vi "pharmaBot_v0.019.vi"() -> ()   [LabVIEW 2015] (continued)
  n42 = control-ref of="memtest 1"() -> (w236:refnum<vi>)
  n43 = control-ref of="cell stats"() -> (w235:refnum<vi>)
  n44 = control-ref of="Ra 1"() -> (w234:refnum<vi>)
  n45 = control-ref of="Ra 2"() -> (w233:refnum<vi>)
  n46 = control-ref of="Cm 1"() -> (w232:refnum<vi>)
  n47 = control-ref of="Cm 2"() -> (w231:refnum<vi>)
  n48 = control-ref of="Iholding 2"() -> (w230:refnum<vi>)
  n49 = control-ref of="P2"() -> (w229:refnum<vi>)
  n50 = control-ref of="Iholding 1"() -> (w228:refnum<vi>)
  n51 = control-ref of="P1"() -> (w227:refnum<vi>)
  n52 = control-ref of="channels to initialize"() -> (w226:refnum<vi>)
  n53 = control-ref of="Multiclamp Handle"() -> (w225:refnum<vi>)
  n54 = control-ref of="mclamp cluster"() -> (w224:refnum<vi>)
  n55 = control-ref of="manip 1 on"() -> (w223:refnum<vi>)
  n56 = control-ref of="manip 2 on"() -> (w222:refnum<vi>)
  n57 = control-ref of="daq_do 2"() -> (w244:refnum<vi>)
  n58 = control-ref of="daq_do 1"() -> (w243:refnum<vi>)
  n59 = control-ref of="NH method"() -> (w179:refnum<vi>)
  n60 = control-ref of="depth"() -> (w178:refnum<vi>)
  n61 = control-ref of="NH R"() -> (w177:refnum<vi>)
  n62 = control-ref of="start GS time 1"() -> (w176:refnum<vi>)
  n63 = control-ref of="max steps to take"() -> (w175:refnum<vi>)
  n64 = control-ref of="Pipette broken threshold (MOhms)"() -> (w173:refnum<vi>)
  n65 = control-ref of="Extra threshold (MOhms)"() -> (w172:refnum<vi>)
  n66 = control-ref of="max hunt distance (um)"() -> (w171:refnum<vi>)
  n67 = control-ref of="Neuron Detection Threshold (MOhms)"() -> (w170:refnum<vi>)
  n68 = control-ref of="hunt pressure (mBar)"() -> (w169:refnum<vi>)
  n69 = control-ref of="NH step size (steps)"() -> (w168:refnum<vi>)
  n70 = control-ref of="current cell 2"() -> (w167:refnum<vi>)
  n71 = control-ref of="cells (image px)"() -> (w166:refnum<vi>)
  n72 = control-ref of="current stage pos (steps)"() -> (w165:refnum<vi>)
  n73 = control-ref of="previous time in"() -> (w164:refnum<vi>)
  n74 = control-ref of="current cell 1"() -> (w162:refnum<vi>)
  n75 = control-ref of="breakin counter 1"() -> (w161:refnum<vi>)
  n76 = control-ref of="MAX Break In Pressure (mbar)"() -> (w160:refnum<vi>)
  n77 = control-ref of="vhold applied?"() -> (w159:refnum<vi>)
  n78 = control-ref of="time"() -> (w158:refnum<vi>)
  n79 = control-ref of="GS R"() -> (w157:refnum<vi>)
  n80 = control-ref of="Vholding (mV) 1"() -> (w156:refnum<vi>)
  n81 = control-ref of="GS timeout (adjusted)"() -> (w155:refnum<vi>)
  n82 = control-ref of="GS timeout (s)"() -> (w154:refnum<vi>)
  n83 = control-ref of="clean bath 2 detected"() -> (w153:refnum<vi>)
  n84 = control-ref of="wash bath 2 detected"() -> (w151:refnum<vi>)
  n85 = control-ref of="wash bath 1 detected"() -> (w150:refnum<vi>)
  n86 = control-ref of="clean bath 1 detected"() -> (w149:refnum<vi>)
  n87 = control-ref of="cleaning status"() -> (w148:refnum<vi>)
  n88 = control-ref of="Wash step (time [s], value [mBar]) actual"() -> (w147:refnum<vi>)
  n89 = control-ref of="Cleaning step (time [s], value [mBar]) actual"() -> (w146:refnum<vi>)
  n90 = control-ref of="pipette score"() -> (w240:refnum<vi>)
  n91 = control-ref of="tip found?"() -> (w241:refnum<vi>)
  n92 = control-ref of="pre-clean"() -> (w145:refnum<vi>)
  n93 = control-ref of="no cell tracker XY zero adjustment (px) (pipette 1 and 2)"() -> (w144:refnum<vi>)
  n94 = control-ref of="cell tracker XY zero adjustment (pipette 1)"() -> (w143:refnum<vi>)
  n95 = control-ref of="pipette template threshold"() -> (w142:refnum<vi>)
  n96 = control-ref of="screen tip location (px)"() -> (w141:refnum<vi>)
  n97 = control-ref of="manip 2 position"() -> (w139:refnum<vi>)
  n98 = control-ref of="manip 1 position"() -> (w138:refnum<vi>)
  n99 = control-ref of="pipette match score"() -> (w137:refnum<vi>)
  n100 = control-ref of="solver_name"() -> (w136:refnum<vi>)
  n101 = control-ref of="tip found 1"() -> (w135:refnum<vi>)
  n102 = control-ref of="cell match score"() -> (w134:refnum<vi>)
  n103 = control-ref of="corrective pipette move"() -> (w133:refnum<vi>)
  n104 = control-ref of="cell found 1"() -> (w132:refnum<vi>)
  n105 = control-ref of="corrective stage move"() -> (w131:refnum<vi>)
  n106 = control-ref of="multiclamp on"() -> (w130:refnum<vi>)
  n107 = control-ref of="skip to successful breakin\n or Cell Attached Protocol"() -> (w129:refnum<vi>)
  n108 = control-ref of="skip gigasealing"() -> (w127:refnum<vi>)
  n109 = control-ref of="cell autofocus"() -> (w126:refnum<vi>)
  n110 = control-ref of="successful breakin 1"() -> (w125:refnum<vi>)
  n111 = control-ref of="User OK"() -> (w124:refnum<vi>)
  n112 = control-ref of="pipette autofocus"() -> (w123:refnum<vi>)
  n113 = control-ref of="skip to unsuccessful breakin"() -> (w122:refnum<vi>)
  n114 = control-ref of="skip hunting"() -> (w121:refnum<vi>)
  n115 = control-ref of="clampex control?"() -> (w120:refnum<vi>)
  n116 = control-ref of="Data log location"() -> (w119:refnum<vi>)
  n117 = control-ref of="Saving to... 1"() -> (w118:refnum<vi>)
  n118 = control-ref of="subtract from distToDescend (steps)"() -> (w117:refnum<vi>)
  n119 = control-ref of="trial data saved"() -> (w115:refnum<vi>)
  n120 = control-ref of="multiclamp control?"() -> (w114:refnum<vi>)
  n121 = control-ref of="simultaneous WC"() -> (w113:refnum<vi>)
  n122 = control-ref of="Sampling Freq (Hz)"() -> (w112:refnum<vi>)
  n123 = control-ref of="dual patch cluster"() -> (w111:refnum<vi>)
  n124 = control-ref of="gigasealing options"() -> (w110:refnum<vi>)
  n125 = control-ref of="Select cells based on proximity (multi patch)"() -> (w109:refnum<vi>)
  n126 = control-ref of="NH wait time (ms)"() -> (w108:refnum<vi>)
  n127 = control-ref of="pressure box 1"() -> (w107:refnum<vi>)
  n128 = control-ref of="wash bath loc 2"() -> (w106:refnum<vi>)
  n129 = control-ref of="cleaning bath loc 2"() -> (w105:refnum<vi>)
  n130 = control-ref of="loc above baths 2"() -> (w103:refnum<vi>)
  n131 = control-ref of="wash bath loc 1"() -> (w102:refnum<vi>)
  n132 = control-ref of="cleaning bath loc 1"() -> (w101:refnum<vi>)
  n133 = control-ref of="loc above baths 1"() -> (w100:refnum<vi>)
  n134 = control-ref of="Jumper Position o-C"() -> (w99:refnum<vi>)
  n135 = control-ref of="Jumper Position C-o"() -> (w98:refnum<vi>)
  n136 = control-ref of="Jumper Position C-B"() -> (w97:refnum<vi>)
  n137 = control-ref of="Jumper Position B-C"() -> (w96:refnum<vi>)
  n138 = control-ref of="Jumper Position B-A"() -> (w95:refnum<vi>)
  n139 = control-ref of="Jumper Position A-B"() -> (w94:refnum<vi>)
  n140 = control-ref of="Jumper Position A-o"() -> (w93:refnum<vi>)
  n141 = control-ref of="Jumper Position o-A"() -> (w91:refnum<vi>)
  n142 = control-ref of="Jumper Position C"() -> (w90:refnum<vi>)
  n143 = control-ref of="Jumper Position B"() -> (w89:refnum<vi>)
  n144 = control-ref of="Jumper Position A"() -> (w88:refnum<vi>)
  n145 = control-ref of="Experiment Safe Position"() -> (w87:refnum<vi>)
  n146 = control-ref of="Jumper Safe Position"() -> (w86:refnum<vi>)
  n147 = control-ref of="Jumper Position o-C Set"() -> (w85:refnum<vi>)
  n148 = control-ref of="Jumper Position C-B Set"() -> (w84:refnum<vi>)
  n149 = control-ref of="Jumper Position B-C Set"() -> (w83:refnum<vi>)
  n150 = control-ref of="Jumper Position B-A Set"() -> (w82:refnum<vi>)
  n151 = control-ref of="Jumper Position A-B Set"() -> (w81:refnum<vi>)
  n152 = control-ref of="Jumper Position A-o Set"() -> (w79:refnum<vi>)
  n153 = control-ref of="Jumper Position o-A Set"() -> (w78:refnum<vi>)
  n154 = control-ref of="Jumper Position C Set"() -> (w77:refnum<vi>)
  n155 = control-ref of="Jumper Position B Set"() -> (w76:refnum<vi>)
  n156 = control-ref of="Jumper Position C-o Set"() -> (w75:refnum<vi>)
  n157 = control-ref of="Jumper Position A Set"() -> (w74:refnum<vi>)
  n158 = control-ref of="Experiment Safe Position Set"() -> (w73:refnum<vi>)
  n159 = control-ref of="Jumper Safe Position Set"() -> (w72:refnum<vi>)
  n160 = control-ref of="Vholding (mV) 2"() -> (w71:refnum<vi>)
  n161 = control-ref of="cleaning status 2"() -> (w70:refnum<vi>)
  n162 = control-ref of="trial data saved 2"() -> (w68:refnum<vi>)
  n163 = control-ref of="NH R 2"() -> (w67:refnum<vi>)
  n164 = control-ref of="cell tracker XY zero adjustment (pipette 2)"() -> (w66:refnum<vi>)
  n165 = control-ref of="depth 2"() -> (w65:refnum<vi>)
  n166 = control-ref of="GS R 2"() -> (w64:refnum<vi>)
  n167 = control-ref of="time 2"() -> (w63:refnum<vi>)
  n168 = control-ref of="breakin counter 2"() -> (w62:refnum<vi>)
  n169 = control-ref of="pipette offset (mV) 2"() -> (w61:refnum<vi>)
  n170 = control-ref of="Saving to... 2"() -> (w60:refnum<vi>)
  n171 = control-ref of="successful breakin 2"() -> (w59:refnum<vi>)
  n172 = control-ref of="cell found 2"() -> (w57:refnum<vi>)
  n173 = control-ref of="tip found 2"() -> (w56:refnum<vi>)
  n174 = control-ref of="GS timeout (adjusted) 2"() -> (w55:refnum<vi>)
  n175 = control-ref of="cell tracking box (px) 2"() -> (w54:refnum<vi>)
  n176 = control-ref of="vhold applied? 2"() -> (w53:refnum<vi>)
  n177 = control-ref of="start GS time 2"() -> (w52:refnum<vi>)
  n178 = control-ref of="screen tip location (px) 2"() -> (w51:refnum<vi>)
  n179 = control-ref of="initial memtest inputs"() -> (w50:refnum<vi>)
  n180 = control-ref of="Memtest inputs"() -> (w49:refnum<vi>)
  n181 = control-ref of="positions"() -> (w5:refnum<vi>)
  n182 = control-ref of="transforms"() -> (w47:refnum<vi>)
  n183 = control-ref of="cam info out"() -> (w46:refnum<vi>)
  n184 = control-ref of="cell diameter (px)"() -> (w45:refnum<vi>)
  n185 = control-ref of="camera type"() -> (w44:refnum<vi>)
  n186 = control-ref of="Adjust exposure (ms)"() -> (w43:refnum<vi>)
  n187 = control-ref of="Range"() -> (w42:refnum<vi>)
  n188 = control-ref of="Distances"() -> (w41:refnum<vi>)
  n189 = control-ref of="Manip 2 Angle [deg]"() -> (w40:refnum<vi>)
  n190 = control-ref of="Manip 2 Distance [mm]"() -> (w39:refnum<vi>)
  n191 = control-ref of="step distance (steps) safe space"() -> (w38:refnum<vi>)
  n192 = control-ref of="Patched Cell Value"() -> (w37:refnum<vi>)
  n193 = control-ref of="Manip 1 Angle [deg]"() -> (w35:refnum<vi>)
  n194 = control-ref of="Manip 1 Distance [mm]"() -> (w34:refnum<vi>)
  n195 = control-ref of="pipette 2 template"() -> (w33:refnum<vi>)
  n196 = control-ref of="pipette 2 mask"() -> (w32:refnum<vi>)
  n197 = control-ref of="temp pipette 2 template location"() -> (w31:refnum<vi>)
  n198 = control-ref of="pipette 1 mask"() -> (w30:refnum<vi>)
  n199 = control-ref of="temp pipette 1 template location"() -> (w29:refnum<vi>)
  n200 = control-ref of="pipette 1 template"() -> (w28:refnum<vi>)
  n201 = control-ref of="nWC"() -> (w27:refnum<vi>)
  n202 = control-ref of="nGS"() -> (w26:refnum<vi>)
  n203 = control-ref of="nAttempts"() -> (w25:refnum<vi>)
  n204 = control-ref of="Calibrate:"() -> (w23:refnum<vi>)
  n205 = control-ref of="Human in Situ"() -> (w22:refnum<vi>)
  n206 = control-ref of="In Process Calibration?"() -> (w21:refnum<vi>)
  n207 = control-ref of="Robotic Break-In?"() -> (w20:refnum<vi>)
  n208 = control-ref of="Vision Fix"() -> (w19:refnum<vi>)
  n209 = control-ref of="Patched Cell Index"() -> (w18:refnum<vi>)
  n210 = control-ref of="Save Resistance"() -> (w17:refnum<vi>)
  n211 = control-ref of="Saved Pipette Resistance"() -> (w16:refnum<vi>)
  n212 = control-ref of="cells selected"() -> (w15:refnum<vi>)
  n213 = control-ref of="cells left"() -> (w14:refnum<vi>)
  n214 = control-ref of="current stage location (px)"() -> (w13:refnum<vi>)
  n215 = control-ref of="current pipette locations (px)"() -> (w12:refnum<vi>)
  n216 = control-ref of="current cell locations (px)"() -> (w11:refnum<vi>)
  n217 = control-ref of="current park plane z (px)"() -> (w10:refnum<vi>)
  n218 = control-ref of="park plane z (px)"() -> (w9:refnum<vi>)
  n219 = control-ref of="save path"() -> (w242:refnum<vi>)
  n220 = Build Array(w244, w243, w242, w241, w240, w239, w238, w237, w236, w235) -> (w190:refnum<vi>[])
  n221 = Build Array(w234, w233, w232, w231, w230, w229, w228, w227, w226, w225, w224) -> (w189:refnum<vi>[])
  n222 = Build Array(w223, w222, w221, w220, w219, w218, w217, w216, w215, w214, w213) -> (w188:refnum<vi>[])
  n223 = Build Array(w162, w161, w160, w159, w158, w157, w156, w155, w154, w153) -> (w152:refnum<vi>[])
  n224 = Build Array(w201, w200, w199, w198, w197, w196, w195, w194, w193, w192, w191) -> (w186:refnum<vi>[])
  n225 = Build Array(w185, w184, w183, w182, w181, w180, w179, w178, w177, w176, w175) -> (w174:refnum<vi>[])
  n226 = Build Array(w173, w172, w171, w170, w169, w168, w167, w166, w165, w164) -> (w163:refnum<vi>[])
  n227 = Build Array(w212, w211, w210, w209, w208, w207, w206, w205, w204, w203, w202) -> (w187:refnum<vi>[])
  n228 = Build Array(w151, w150, w149, w148, w147, w146, w145, w144, w143, w142, w141) -> (w140:refnum<vi>[])
  n229 = Build Array(w68, w67, w66, w65, w64, w63, w62, w61, w60, w59) -> (w58:refnum<vi>[])
  n230 = Build Array(w79, w78, w77, w76, w75, w74, w73, w72, w71, w70) -> (w69:refnum<vi>[])
  n231 = Build Array(w57, w56, w55, w54, w53, w52, w51, w50, w49, w6, w5) -> (w48:refnum<vi>[])
  n232 = Build Array(w47, w46, w45, w44, w43, w42, w41, w40, w39, w38, w37) -> (w36:refnum<vi>[])
  n233 = Build Array(w23, w22, w21, w20, w19, w18, w17, w16, w15, w14, w13, w12, w11, w10, w9) -> (w8:refnum<vi>[])
  n234 = Build Array(w127, w126, w125, w124, w123, w122, w121, w120, w119, w118, w117) -> (w116:refnum<vi>[])
  n235 = Build Array(w91, w90, w89, w88, w87, w86, w85, w84, w83, w82, w81) -> (w80:refnum<vi>[])
  n236 = Build Array(w35, w34, w33, w32, w31, w30, w29, w28, w27, w26, w25) -> (w24:refnum<vi>[])
  n237 = Build Array(w115, w114, w113, w112, w111, w110, w109, w108, w107, w106, w105) -> (w104:refnum<vi>[])
  n238 = Build Array(w103, w102, w101, w100, w99, w98, w97, w96, w95, w94, w93) -> (w92:refnum<vi>[])
  n239 = Build Array(w139, w138, w137, w136, w135, w134, w133, w132, w131, w130, w129) -> (w128:refnum<vi>[])
  n240 = Build Array (concatenate)(w190, w189, w188, w187, w186, w174, w163, w152, w140, w128, w116, w104, w92, w80, w69, w58, w48, w36, w24, w8) -> (→"allMainVIcontrols":refnum<vi>[])
  n241 = control-ref of="gigasealing options 2"() -> ()  [unwired: 1 out]
  n242 = control-ref of="cell tracker"() -> (w538:refnum<vi>)
  n243 = control-ref of="skip gigasealing"() -> (w539:refnum<vi>)
  n244 = control-ref of="clampex control?"() -> (w620:refnum<vi>)
  n245 = control-ref of="demo clean"() -> (w619:refnum<vi>)
  n246 = control-ref of="skip hunting"() -> (w618:refnum<vi>)
  n247 = control-ref of="multiclamp control?"() -> (w617:refnum<vi>)
  n248 = control-ref of="corrective pipette move"() -> (w616:refnum<vi>)
  n249 = control-ref of="corrective stage move"() -> (w615:refnum<vi>)
  n250 = control-ref of="demo daq?"() -> (w614:refnum<vi>)
  n251 = control-ref of="skip to unsuccessful breakin"() -> (w613:refnum<vi>)
  n252 = control-ref of="skip to successful breakin\n or Cell Attached Protocol"() -> (w612:refnum<vi>)
  n253 = control-ref of="successful breakin 1"() -> (w385:refnum<vi>)
  n254 = Bundle(cluster=T48 {"clampex control?"=refnum, "demo clean"=refnum, "skip hunting"=refnum, "skip gigasealing"=refnum, "multiclamp control?"=refnum, "corrective pipette move"=refnum, "corrective stage move"=refnum, "cell tracker"=refnum, "demo daq?"=refnum, "skip to unsuccessful breakin"=refnum, "skip to successful breakin"=refnum, "successful breakin"=refnum} ("state UI indiv"), "clampex control?"=w620, "demo clean"=w619, "skip hunting"=w618, "skip gigasealing"=w539, "multiclamp control?"=w617, "corrective pipette move"=w616, "corrective stage move"=w615, "cell tracker"=w538, "demo daq?"=w614, "skip to unsuccessful breakin"=w613, "skip to successful breakin"=w612, "successful breakin"=w385) -> (w386:T48)
  n255 = control-ref of="pressure box 1"() -> (w380:refnum<vi>)
  n256 = control-ref of="vertical z dist (vertical rel only)  (px)"() -> (w430:refnum<vi>)
  n257 = control-ref of="current cell 1"() -> (w480:refnum<vi>)
  n258 = control-ref of="NH step size (steps)"() -> (w568:refnum<vi>)
  n259 = control-ref of="hunt pressure (mBar)"() -> (w567:refnum<vi>)
  n260 = control-ref of="distToDescend (steps)"() -> (w566:refnum<vi>)
  n261 = control-ref of="above dist (approach above only) (steps)"() -> (w565:refnum<vi>)
  n262 = control-ref of="initial positioning"() -> (w564:refnum<vi>)
  n263 = control-ref of="subtract from distToDescend (steps)"() -> (w563:refnum<vi>)
  n264 = control-ref of="NEURON HUNTING MONITOR"() -> (w562:refnum<vi>)
  n265 = control-ref of="Memtest inputs"() -> (w561:refnum<vi>)
  n266 = control-ref of="max hunt distance (um)"() -> (w529:refnum<vi>)
  n267 = control-ref of="Neuron Detection Threshold (MOhms)"() -> (w528:refnum<vi>)
  n268 = control-ref of="Pipette broken threshold (MOhms)"() -> (w527:refnum<vi>)
  n269 = control-ref of="gross descent pressure (mBar)"() -> (w526:refnum<vi>)
  n270 = control-ref of="Extra threshold (MOhms)"() -> (w525:refnum<vi>)
  n271 = control-ref of="NH wait time (ms)"() -> (w409:refnum<vi>)
  n272 = control-ref of="cell found 1"() -> (w470:refnum<vi>)
  n273 = control-ref of="positions"() -> (w577:refnum<vi>)
  n274 = control-ref of="unpatched cell indices"() -> (w481:refnum<vi>)
  n275 = control-ref of="current cell locations (px)"() -> (w586:refnum<vi>)
  n276 = control-ref of="cells (image px)"() -> (w585:refnum<vi>)
  n277 = control-ref of="current park plane z (px)"() -> (w584:refnum<vi>)
  n278 = control-ref of="current pipette locations (px)"() -> (w543:refnum<vi>)
  n279 = control-ref of="transforms"() -> (w576:refnum<vi>)
  n280 = control-ref of="gross descent pressure (mBar)"() -> (w597:refnum<vi>)
  n281 = control-ref of="NH method"() -> (w375:refnum<vi>)
  n282 = Bundle(cluster=w298, "current cell locations (px)"=w586, "cells (image px)"=w585, "current park plane z (px)"=w584, "gross descent pressure (mBar)"=w597, "positions"=w577, "transforms"=w576, "pressure box"=w380, "current pipette locations (px)"=w543, "unpatched cell indices"=w481, "NH method"=w375, "NH wait time (ms)"=w409) -> (w379:T43)
  n283 = control-ref of="pipette motion"() -> (w335:refnum<vi>)
  n284 = Bundle By Name(cluster=T49 {"NH step size (steps)"=refnum, "hunt pressure (mBar)"=refnum, "distToDescend (steps)"=refnum, "approach above cell (steps)"=refnum, "initial positioning"=refnum, "d(above cell) (steps)"=refnum, "neuron found"=refnum, "NEURON HUNTING MONITOR"=refnum, "Memtest inputs"=refnum, "max hunt distance (um)"=refnum, "Neuron Detection Threshold (MOhms)"=refnum, "Pipette broken threshold (MOhms)"=refnum, "gross descent pressure (mBar)"=refnum, "Extra threshold (MOhms)"=refnum, "current cell"=refnum, "vertical z dist (vertical rel only)  (px)"=refnum} ("positioning + hunting indiv"), "NH step size (steps)"=w568, "hunt pressure (mBar)"=w567, "distToDescend (steps)"=w566, "approach above cell (steps)"=w565, "initial positioning"=w564, "d(above cell) (steps)"=w563, "neuron found"=w470, "NEURON HUNTING MONITOR"=w562, "Memtest inputs"=w561, "max hunt distance (um)"=w529, "Neuron Detection Threshold (MOhms)"=w528, "Pipette broken threshold (MOhms)"=w527, "gross descent pressure (mBar)"=w526, "Extra threshold (MOhms)"=w525, "current cell"=w480, "vertical z dist (vertical rel only)  (px)"=w430) -> (w389:T49)
  n285 = control-ref of="Ra 1"() -> (w376:refnum<vi>)
  n286 = control-ref of="GS timeout (s)"() -> (w611:refnum<vi>)
  n287 = control-ref of="GS timeout (adjusted)"() -> (w610:refnum<vi>)
  n288 = control-ref of="vhold applied?"() -> (w571:refnum<vi>)
  n289 = control-ref of="P1"() -> (w570:refnum<vi>)
  n290 = control-ref of="Iholding 1"() -> (w560:refnum<vi>)
  n291 = control-ref of="start GS time 1"() -> (w559:refnum<vi>)
  n292 = control-ref of="GIGASEALING MONITOR"() -> (w558:refnum<vi>)
  n293 = control-ref of="Vholding (mV) 1"() -> (w542:refnum<vi>)
  n294 = control-ref of="GS extended 1"() -> (w541:refnum<vi>)
  n295 = control-ref of="holding V (mV)"() -> (w428:refnum<vi>)
  n296 = control-ref of="Cm 1"() -> (w377:refnum<vi>)
  n297 = control-ref of="gigasealing options"() -> (w422:refnum<vi>)
  n298 = control-ref of="initialized"() -> (w609:refnum<vi>)
  n299 = control-ref of="Data log location"() -> (w608:refnum<vi>)
  n300 = control-ref of="User OK"() -> (w537:refnum<vi>)
  n301 = control-ref of="mclamp cluster"() -> (w574:refnum<vi>)
  n302 = control-ref of="stage idle?"() -> (w532:refnum<vi>)
  n303 = control-ref of="Multiclamp Handle"() -> (w575:refnum<vi>)
  n304 = control-ref of="stop"() -> (w436:refnum<vi>)
  n305 = control-ref of="dual patch cluster"() -> (w413:refnum<vi>)
  n306 = control-ref of="stop memtest"() -> (w415:refnum<vi>)
  n307 = control-ref of="simultaneous WC"() -> (w412:refnum<vi>)
  n308 = control-ref of="Select cells based on proximity (multi patch)"() -> (w410:refnum<vi>)
  n309 = control-ref of="Validate"() -> (w1:refnum<vi>)
  n310 = control-ref of="Terminate Experiment"() -> (w4:refnum<vi>)
  n311 = control-ref of="dual WC keep going"() -> (w390:refnum<vi>)
  n312 = control-ref of="HEK/slice options"() -> (w381:refnum<vi>)
  n313 = Bundle(cluster=w299, "GS timeout (s)"=w611, "GS timeout (adjusted)"=w610, "vhold applied?"=w571, "pipette resistance"=w570, "Iholding"=w560, "start GS time"=w559, "GIGASEALING MONITOR"=w558, "current Vholding (mV)"=w542, "GS extended"=w541, "holding V (mV)"=w428, "gigasealing options"=w422, "Cm 1"=w377, "Ra 1"=w376) -> (w423:T44)
  n314 = flat-sequence {
    tunnel: [w706] -> w393
    tunnel: w393 -> [w720]
    tunnel: [w720] -> w392
    tunnel: w258 -> [w715]
    tunnel: w259 -> [w710]
    frame #0 {
      n315 = local read "initial memtest inputs"() -> (w705:T29)
      n316 = invoke on="Manip 3 Calibrated" class="Bool (strict)" method="Reinit To Default"() -> ()  [unwired: 3 in, 3 out]
      n317 = invoke on="Manip 2 Calibrated" class="Bool (strict)" method="Reinit To Default"() -> ()  [unwired: 3 in, 3 out]
      n318 = invoke on="nAttempts" class="DigNum (strict)" method="Reinit To Default"() -> ()  [unwired: 3 in, 3 out]
      n319 = invoke on="nGS" class="DigNum (strict)" method="Reinit To Default"() -> ()  [unwired: 3 in, 3 out]
      n320 = invoke on="Manip 1 Calibrated" class="Bool (strict)" method="Reinit To Default"() -> ()  [unwired: 3 in, 3 out]
      n321 = local write "Calibration Protocol"(T7."Init" ("Calibration Protocol")) -> ()
      n322 = local write "Memtest inputs"(w705) -> ()
      n323 = invoke on="Manip 4 Calibrated" class="Bool (strict)" method="Reinit To Default"() -> (error out=w706:errorcluster)  [unwired: 3 in, 2 out]
      n324 = invoke on="Pipette is in Focus?" class="Bool (strict)" method="Reinit To Default"() -> ()  [unwired: 3 in, 3 out]
      n325 = invoke on="Stage zeroed?" class="Bool (strict)" method="Reinit To Default"() -> ()  [unwired: 3 in, 3 out]
      n326 = invoke on="nWC" class="DigNum (strict)" method="Reinit To Default"() -> ()  [unwired: 3 in, 3 out]
    }
    frame #1 {
      w709 = FALSE
      n327 = local read "Stage Shift (steps)"() -> (w719:dbl)
      n328 = local write "Jump o-C Good?"(w709) -> ()
      n329 = local write "Jump C-o Good?"(w709) -> ()
      n330 = local write "Jump C-B Good?"(w709) -> ()
      n331 = Negate(x=w719) -> (-x=w717:dbl)
      n332 = Divide(x=w717, y=10.0) -> (x/y=w716:dbl)
      n333 = property on="Next Stage and Pipette Z Location" class="Slide (strict)"("Scale.Maximum"=w716) -> ()  [unwired: 2 in, 2 out]
      n334 = local read "Valve1 Connected"() -> (w708:bool)
      n335 = local write "Jump Pos o-C"(w709) -> ()
      n336 = local write "Jump Pos C-o"(w709) -> ()
      n337 = local write "Jump Pos C-B"(w709) -> ()
      n338 = local write "Jump Pos B-A"(w709) -> ()
      n339 = local read "Valve2 Connected"() -> (w707:bool)
      n340 = local write "V1-Changing"(FALSE ("Valve1-Changing")) -> ()
      n341 = case shown="True" w707 {
        tunnel: [u16 0 ("ValveSetTo") w723] -> w711
        tunnel: w710 -> [_ w722]
        frame False {
        }
        frame True {
          n342 = call "initializeValveDigital-v02.vi"("daq_do"=w722) -> ("ValveSetTo"=w723:u16)  [unwired: 10 in]
        }
      }
      n343 = case shown="True" w708 {
        tunnel: w715 -> [_ w726]
        tunnel: [u16 0 ("ValveSetTo") w725] -> w714
        frame False {
        }
        frame True {
          n344 = call "initializeValveDigital-v02.vi"("daq_do"=w726) -> ("ValveSetTo"=w725:u16)  [unwired: 10 in]
        }
      }
      n345 = local write "V2-Changing"(FALSE ("Valve1-Changing")) -> ()
      n346 = local write "Jump B-C Good?"(w709) -> ()
      n347 = local write "Jump B-A Good?"(w709) -> ()
      n348 = local write "Jump A-B Good?"(w709) -> ()
      n349 = local write "Jump A-o Good?"(w709) -> ()
      n350 = local write "Jump o-A Good?"(w709) -> ()
      n351 = local write "Experiment Safe"(w709) -> ()
      n352 = local write "Jumper Safe"(w709) -> ()
      n353 = local write "Valve2"(w711) -> ()
      n354 = local write "V2-State"(w711) -> ()
      n355 = local write "Valve1"(w714) -> ()
      n356 = call "initializeValveSerial-v01.vi"() -> ()  [unwired: 9 in, 3 out]
      n357 = local write "V1-State"(w714) -> ()
      n358 = local write "Jump Pos A-B"(w709) -> ()
      n359 = local write "Jump Pos A-o"(w709) -> ()
      n360 = local write "Jump Pos o-A"(w709) -> ()
      n361 = local write "Pos A"(w709) -> ()
      n362 = local write "Jump Pos B-C"(w709) -> ()
      n363 = local write "Pos C"(w709) -> ()
      n364 = local write "Pos B"(w709) -> ()
    }
  }
  n365 = Bundle(cluster=T39 {"initialized"=refnum, "Data log location"=refnum, "Multiclamp Handle"=refnum, "mclamp cluster"=refnum, "User OK"=refnum, "stage idle?"=refnum, "stop"=refnum, "pipette motion"=refnum, "stop memtest"=refnum, "dual patch cluster"=refnum, "simultaneous WC"=refnum, "Select cells based on proximity (multi patch)"=refnum, "dual WC keep going"=refnum, "HEK/slice options"=refnum, "Terminate Experiment"=refnum, "Validate"=refnum} ("miscCommon"), "initialized"=w609, "Data log location"=w608, "Multiclamp Handle"=w575, "mclamp cluster"=w574, "User OK"=w537, "stage idle?"=w532, "stop"=w436, "pipette motion"=w335, "stop memtest"=w415, "dual patch cluster"=w413, "simultaneous WC"=w412, "Select cells based on proximity (multi patch)"=w410, "dual WC keep going"=w390, "HEK/slice options"=w381, "Terminate Experiment"=w4, "Validate"=w1) -> (w391:T39)
  n366 = control-ref of="pipette offset (mV)"() -> (w607:refnum<vi>)
  n367 = control-ref of="time"() -> (w582:refnum<vi>)
  n368 = control-ref of="depth"() -> (w581:refnum<vi>)
  n369 = control-ref of="NH R"() -> (w580:refnum<vi>)
  n370 = control-ref of="GS R"() -> (w579:refnum<vi>)
  n371 = control-ref of="Command pressure (mBar) 1"() -> (w573:refnum<vi>)
  n372 = local read "daq_ao"() -> (w557:tag)
  n373 = local read "daq_ai"() -> (w556:tag)
  n374 = control-ref of="Saving to... 1"() -> (w321:refnum<vi>)
  n375 = control-ref of="state times 1"() -> (w555:refnum<vi>)
  n376 = control-ref of="Sampling Freq (Hz)"() -> (w320:refnum<vi>)
  n377 = local read "daq_do 2"() -> (w319:tag)
  n378 = control-ref of="Robotic Break-In?"() -> (w314:refnum<vi>)
  n379 = control-ref of="pipette 1 broken - abort!"() -> (w554:refnum<vi>)
  n380 = control-ref of="trial data saved"() -> (w553:refnum<vi>)
  n381 = control-ref of="state list manip 1"() -> (w552:refnum<vi>)
  n382 = control-ref of="stage reservation options"() -> (w531:refnum<vi>)
  n383 = control-ref of="retract distance (um)"() -> (w524:refnum<vi>)
  n384 = local read "daq_do 1"() -> (w318:tag)
  n385 = control-ref of="Human Control Done"() -> (w312:refnum<vi>)
  n386 = local read "daq_ao 2"() -> (w317:tag)
  n387 = control-ref of="V1-State"() -> (w311:refnum<vi>)
  n388 = control-ref of="P1 state"() -> (w290:refnum<vi>)
  n389 = control-ref of="P2 state"() -> (w291:refnum<vi>)
  n390 = control-ref of="In Process Calibration?"() -> (w313:refnum<vi>)
  n391 = control-ref of="V2-State"() -> (w310:refnum<vi>)
  n392 = control-ref of="Human in Situ"() -> (w316:refnum<vi>)
  n393 = control-ref of="State to advance to after Human Control"() -> (w292:refnum<vi>)
  n394 = control-ref of="Break-In Counter"() -> (w315:refnum<vi>)
  n395 = control-ref of="init tracker success"() -> (w593:refnum<vi>)
  n396 = control-ref of="run tracker success"() -> (w592:refnum<vi>)
  n397 = control-ref of="tracking"() -> (w591:refnum<vi>)
  n398 = control-ref of="exit tracker success"() -> (w590:refnum<vi>)
  n399 = control-ref of="current pipette locations (px)"() -> (w589:refnum<vi>)
  n400 = control-ref of="cell image size (px)"() -> (w588:refnum<vi>)
  n401 = control-ref of="pipette match score"() -> (w587:refnum<vi>)
  n402 = control-ref of="cell match score"() -> (w569:refnum<vi>)
  n403 = control-ref of="P1 state"() -> (w306:refnum<vi>)
  n404 = control-ref of="P2 state"() -> (w307:refnum<vi>)
  n405 = control-ref of="cell tracker init error out"() -> (w540:refnum<vi>)
  n406 = control-ref of="state times 2"() -> (w507:refnum<vi>)
  n407 = control-ref of="pipette 2 broken - abort!"() -> (w506:refnum<vi>)
  n408 = control-ref of="trial data saved 2"() -> (w505:refnum<vi>)
  n409 = control-ref of="state list manip 2"() -> (w504:refnum<vi>)
  n410 = control-ref of="time 2"() -> (w492:refnum<vi>)
  n411 = control-ref of="depth 2"() -> (w491:refnum<vi>)
  n412 = control-ref of="NH R 2"() -> (w490:refnum<vi>)
  n413 = control-ref of="GS R 2"() -> (w489:refnum<vi>)
  n414 = control-ref of="Command pressure (mBar) 2"() -> (w487:refnum<vi>)
  n415 = control-ref of="pipette offset (mV) 2"() -> (w488:refnum<vi>)
  n416 = control-ref of="Saving to... 2"() -> (w305:refnum<vi>)
  n417 = Bundle(cluster=w295, "init tracker success"=w593, "run tracker success"=w592, "tracking"=w591, "exit tracker success"=w590, "init error out"=w540, "current pipette locations (px)"=w589, "cell image size (px)"=w588, "pipette match score"=w587, "cell match score"=w569) -> (w455:T40)
  n418 = control-ref of="pipette_px_onscreen"() -> (w546:refnum<vi>)
  n419 = control-ref of="pipette template threshold"() -> (w454:refnum<vi>)
  n420 = control-ref of="pipette centroid array"() -> (w451:refnum<vi>)
  n421 = control-ref of="cell length (px)"() -> (w438:refnum<vi>)
  n422 = control-ref of="centroid_px"() -> (w547:refnum<vi>)
  n423 = control-ref of="pipette_tracking_quality"() -> (w545:refnum<vi>)
  n424 = control-ref of="cell_tracking_quality"() -> (w544:refnum<vi>)
  n425 = control-ref of="cell centroid array"() -> (w452:refnum<vi>)
  n426 = control-ref of="solver_beta"() -> (w606:refnum<vi>)
  n427 = control-ref of="solver_kappa"() -> (w605:refnum<vi>)
  n428 = control-ref of="shear_angle"() -> (w604:refnum<vi>)
  n429 = control-ref of="solver_gamma"() -> (w603:refnum<vi>)
  n430 = control-ref of="template_window"() -> (w602:refnum<vi>)
  n431 = control-ref of="debug_mode"() -> (w601:refnum<vi>)
  n432 = control-ref of="psf_sigma"() -> (w600:refnum<vi>)
  n433 = control-ref of="solver_name"() -> (w599:refnum<vi>)
  n434 = control-ref of="cell found 2"() -> (w511:refnum<vi>)
  n435 = control-ref of="tip found 2"() -> (w510:refnum<vi>)
  n436 = control-ref of="cell tracking box (px) 2"() -> (w509:refnum<vi>)
  n437 = Bundle(cluster="misc indiv", "pipette offset (mV)"=w607, "time"=w582, "depth"=w581, "NH R"=w580, "GS R"=w579, "Command pressure (mBar)"=w573, "daq_ao"=w557, "daq_ai"=w556, "state times"=w555, "pipette broken - abort!"=w554, "trial data saved"=w553, "state list"=w552, "stage reservation options"=w531, "retract distance (um)"=w524, "Saving to..."=w321, "Sampling Freq (Hz)"=w320, "daq_do 2"=w319, "daq_do 1"=w318, "daq_ao 2"=w317, "Human in Situ"=w316, "Break-In Counter"=w315, "Robotic Break-In?"=w314, "In Process Calibration?"=w313, "Human Control Done"=w312, "V1-State"=w311, "V2-State"=w310, "State to advance to after Human Control"=w292, "other state ref"=w291, "state ref"=w290) -> (w309:T1)
  n438 = Bundle By Name(cluster=w309, "state times"=w507, "pipette broken - abort!"=w506, "trial data saved"=w505, "state list"=w504, "time"=w492, "depth"=w491, "NH R"=w490, "GS R"=w489, "Command pressure (mBar)"=w487, "pipette offset (mV)"=w488, "state ref"=w307, "Saving to..."=w305, "other state ref"=w306) -> (w308:T1)
  n439 = Bundle(cluster=w296, "solver_beta"=w606, "solver_kappa"=w605, "shear_angle"=w604, "solver_gamma"=w603, "template_window"=w602, "debug_mode"=w601, "psf_sigma"=w600, "solver_name"=w599, "centroid_px"=w547, "pipette_px"=w546, "pipette_tracking_quality"=w545, "cell_tracking_quality"=w544, "pipette template threshold"=w454, "cell centroid array"=w452, "pipette centroid array"=w451, "cell length (px)"=w438) -> (w450:T41)
  n440 = control-ref of="cell found 1"() -> (w596:refnum<vi>)
  n441 = control-ref of="tip found 1"() -> (w595:refnum<vi>)
  n442 = control-ref of="cell tracking box (px)"() -> (w594:refnum<vi>)
  n443 = control-ref of="screen tip location (px)"() -> (w551:refnum<vi>)
  n444 = control-ref of="Experimental VI To Run"() -> (w352:refnum<vi>)
  n445 = control-ref of="Project"() -> (w373:refnum<vi>)
  n446 = control-ref of="AnalysisProtocol"() -> (w372:refnum<vi>)
  n447 = control-ref of="PatchSettings"() -> (w371:refnum<vi>)
  n448 = control-ref of="Passage/Age"() -> (w370:refnum<vi>)
  n449 = control-ref of="CellType"() -> (w369:refnum<vi>)
  n450 = control-ref of="Experiment"() -> (w368:refnum<vi>)
  n451 = control-ref of="Conditions"() -> (w367:refnum<vi>)
  n452 = local write "GS extended 2"(w262) -> ()
  n453 = local write "GS extended 1"(w262) -> ()
  n454 = Bundle(cluster=w517, "screen tip location (px)"=w551, "cell found"=w596, "tip found"=w595, "cell tracking box (px)"=w594) -> (w475:T51)
  n455 = Bundle By Name(cluster=w475, "cell found"=w511, "tip found"=w510, "cell tracking box (px)"=w509) -> (w508:T51)
  n456 = control-ref of="cell tracker XY zero adjustment (pipette 1)"() -> (w404:refnum<vi>)
  n457 = control-ref of="no cell tracker XY zero adjustment (px) (pipette 1 and 2)"() -> (w383:refnum<vi>)
  n458 = Bundle(cluster=w297, "Project"=w373, "AnalysisProtocol"=w372, "PatchSettings"=w371, "Passage/Age"=w370, "CellType"=w369, "Experiment"=w368, "Conditions"=w367, "ExperimentVIToRun"=w352) -> (w374:T42)
  n459 = control-ref of="MAX Break In Pressure (mbar)"() -> (w522:refnum<vi>)
  n460 = control-ref of="pre-clean"() -> (w598:refnum<vi>)
  n461 = control-ref of="loc above baths 1"() -> (w550:refnum<vi>)
  n462 = control-ref of="wash bath loc 1"() -> (w549:refnum<vi>)
  n463 = control-ref of="cleaning bath loc 1"() -> (w548:refnum<vi>)
  n464 = control-ref of="cleaning status"() -> (w486:refnum<vi>)
  n465 = control-ref of="avg peak height 1"() -> (w485:refnum<vi>)
  n466 = control-ref of="clean bath 1 detected"() -> (w420:refnum<vi>)
  n467 = control-ref of="wash bath 1 detected"() -> (w419:refnum<vi>)
  n468 = control-ref of="GS extended 2"() -> (w495:refnum<vi>)
  n469 = control-ref of="loc above baths 2"() -> (w516:refnum<vi>)
  n470 = control-ref of="wash bath loc 2"() -> (w515:refnum<vi>)
  n471 = control-ref of="cleaning bath loc 2"() -> (w514:refnum<vi>)
  n472 = control-ref of="cleaning status 2"() -> (w513:refnum<vi>)
  n473 = control-ref of="avg peak height 2"() -> (w512:refnum<vi>)
  n474 = control-ref of="GIGASEALING MONITOR 2"() -> (w503:refnum<vi>)
  n475 = control-ref of="start GS time 2"() -> (w502:refnum<vi>)
  n476 = control-ref of="GS timeout (adjusted) 2"() -> (w501:refnum<vi>)
  n477 = control-ref of="vhold applied? 2"() -> (w500:refnum<vi>)
  n478 = control-ref of="P2"() -> (w499:refnum<vi>)
  n479 = control-ref of="Iholding 2"() -> (w498:refnum<vi>)
  n480 = control-ref of="Vholding (mV) 2"() -> (w496:refnum<vi>)
  n481 = flat-sequence {
    tunnel: [w730] -> w471
    tunnel: w278 -> [_]
    tunnel: [w727] -> w281
    frame #0 {
      w735 = T54 {"slice image"=refnum, "pipette template"=refnum, "found pipette"=refnum, "pipette mask for cell tracker"=refnum, "cell images ref"=refnum}  # images
      n482 = local read "pipette 1 mask for cell tracker"() -> (w731:T10)
      n483 = control-ref of="cell images"() -> (w729:refnum<vi>)
      n484 = local read "pipette 1 template"() -> (w733:T10)
      n485 = local read "found pipette 1"() -> (w732:T10)
      n486 = local read "Slice view"() -> (w734:T10)
      n487 = control-ref of="cam size"() -> (w728:refnum<vi>)
      n488 = Bundle By Name(cluster=w735, "slice image"=w734, "pipette template"=w733, "found pipette"=w732, "cell images ref"=w729, "pipette mask for cell tracker"=w731) -> (w730:T54)
      n489 = property class="Arr (strict)"(reference=w728) -> ("Value"=w727:i32[])  [unwired: 1 in, 2 out]
    }
  }
  n490 = local write "initialized"(w521) -> ()
  n491 = local write "pipette 1 broken - abort!"(w521) -> ()
  n492 = local write "User OK"(w521) -> ()
  n493 = local write "trial data saved"(w521) -> ()
  n494 = local write "multiclamp on"(w521) -> ()
  n495 = local write "stop always"(w521) -> ()
  n496 = local write "stop"(w521) -> ()
  n497 = control-ref of="Jumper Position o-C"() -> (w351:refnum<vi>)
  n498 = control-ref of="Jumper Position C-o"() -> (w350:refnum<vi>)
  n499 = control-ref of="Jumper Position C-B"() -> (w349:refnum<vi>)
  n500 = control-ref of="Jumper Position B-C"() -> (w348:refnum<vi>)
  n501 = control-ref of="Jumper Position B-A"() -> (w347:refnum<vi>)
  n502 = control-ref of="Jumper Position A-B"() -> (w346:refnum<vi>)
  n503 = control-ref of="Jumper Position A-o"() -> (w345:refnum<vi>)
  n504 = control-ref of="Jumper Position o-A"() -> (w344:refnum<vi>)
  n505 = control-ref of="Jumper Position C"() -> (w343:refnum<vi>)
  n506 = control-ref of="Jumper Position B"() -> (w342:refnum<vi>)
  n507 = control-ref of="Jumper Position A"() -> (w341:refnum<vi>)
  n508 = control-ref of="Experiment Safe Position"() -> (w340:refnum<vi>)
  n509 = control-ref of="Jumper Safe Position"() -> (w339:refnum<vi>)
  n510 = control-ref of="manip 1 position"() -> (w530:refnum<vi>)
  n511 = control-ref of="breakin counter 1"() -> (w572:refnum<vi>)
  n512 = Bundle("manip 1 position"=w530, "cell tracker XY zero adjustment (pipette 1)"=w404, "no cell tracker XY zero adjustment (px) (pipette 1 and 2)"=w383) -> (w476:T55)  [unwired: 1 in]
  n513 = Bundle By Name(cluster=w423, "GIGASEALING MONITOR"=w503, "start GS time"=w502, "GS timeout (adjusted)"=w501, "vhold applied?"=w500, "pipette resistance"=w499, "Iholding"=w498, "current Vholding (mV)"=w496, "GS extended"=w495) -> (w497:T44)
  n514 = Bundle(cluster=w426, "pre-clean"=w598, "loc above baths"=w550, "wash bath loc"=w549, "cleaning bath loc"=w548, "cleaning status"=w486, "avg peak height"=w485, "clean bath detected"=w420, "wash bath detected"=w419) -> (w427:T50)
  n515 = Bundle(cluster=w523, "breakin counter"=w572, "MAX Break In Pressure (mbar)"=w522) -> (w477:T52)
  n516 = control-ref of="NEURON HUNTING MONITOR 2"() -> (w494:refnum<vi>)
  n517 = control-ref of="Command pressure (mBar) 2"() -> (w493:refnum<vi>)
  n518 = control-ref of="current cell 2"() -> (w479:refnum<vi>)
  n519 = control-ref of="manip 2 position"() -> (w437:refnum<vi>)
  n520 = control-ref of="clean bath 2 detected"() -> (w425:refnum<vi>)
  n521 = control-ref of="wash bath 2 detected"() -> (w424:refnum<vi>)
  n522 = control-ref of="breakin counter 2"() -> (w418:refnum<vi>)
  n523 = Bundle(cluster=w300, "JumperPos o-C"=w351, "JumperPos C-o"=w350, "JumperPos C-B"=w349, "JumperPos B-C"=w348, "JumperPos B-A"=w347, "JumperPos A-B"=w346, "JumperPos A-o"=w345, "JumperPos o-A"=w344, "JumperPos C"=w343, "JumperPos B"=w342, "JumperPos A"=w341, "ExpSafePos"=w340, "jumperSafePos"=w339) -> (w337:T45)
  n524 = Bundle By Name(cluster=w427, "loc above baths"=w516, "wash bath loc"=w515, "cleaning bath loc"=w514, "cleaning status"=w513, "avg peak height"=w512) -> (w484:T50)
  n525 = local read "pipette 2 mask for cell tracker"() -> (w465:T10)
  n526 = control-ref of="ValidationResults"() -> (w304:refnum<vi>)
  n527 = control-ref of="ValidationPos1"() -> (w303:refnum<vi>)
  n528 = control-ref of="ValidationOutputCluster"() -> (w294:refnum<vi>)
  n529 = control-ref of="ValidationPos2"() -> (w302:refnum<vi>)
  n530 = local write "state times 2"(w263) -> ()
  n531 = local write "state times 1"(w263) -> ()
  n532 = local read "cell tracker"() -> (w261:bool)
  n533 = local write "current cell 2"(w478) -> ()
  n534 = local write "current cell 1"(w478) -> ()
  n535 = Bundle(cluster=T46 {"ValidationResults"=refnum, "ValidationPos1"=refnum, "ValidationPos2"=refnum, "ValidationOutputCluster"=refnum} ("PreviousValidationResults"), "ValidationResults"=w304, "ValidationPos1"=w303, "ValidationPos2"=w302, "ValidationOutputCluster"=w294) -> (w301:T46)
  n536 = Bundle By Name(cluster=w583, "cell tracker common"=w450, "vision common"=w455, "misc common"=w391, "positioning+hunting common"=w379, "ExperimentDescriptors"=w374, "JumperPositions"=w337, "PreviousValidationResults"=w301) -> (w245:T37)
  n537 = control-ref of="successful breakin 2"() -> (w384:refnum<vi>)
  n538 = control-ref of="cell tracker XY zero adjustment (pipette 2)"() -> (w405:refnum<vi>)
  n539 = local read "pipette 2 template"() -> (w469:T10)
  n540 = local read "found pipette 2"() -> (w468:T10)
  n541 = Bundle By Name(cluster=w578, "state UI indiv"=w386, "positioning + hunting indiv"=w389, "gigaseal indiv"=w423, "misc indiv"=w309, "cleaning indiv"=w427, "cell tracker indiv"=w475, "breakin indiv"=w477, "vision indiv"=w476) -> (w246:T34)
  n542 = local write "common controls"(w245) -> ()
  n543 = Bundle By Name(cluster=w246, "cleaning indiv"=w484, "cell tracker indiv"=w508, "misc indiv"=w308, "gigaseal indiv"=w497, "positioning + hunting indiv.NEURON HUNTING MONITOR"=w494, "breakin indiv.breakin counter"=w418, "misc indiv.Command pressure (mBar)"=w493, "positioning + hunting indiv.current cell"=w479, "vision indiv.manip position"=w437, "cleaning indiv.clean bath detected"=w425, "cleaning indiv.wash bath detected"=w424, "vision indiv.cell tracker XY zero adjustment (px)"=w405, "state UI indiv.successful breakin"=w384) -> (w249:T34)
  n544 = Select(t=T17."unreserve after cell found" ("stage reservation options"), s=w261, f=T17."unreserve after gross approach" ("stage reservation options")) -> (s? t:f=w407:T17)
  n545 = local write "stage idle?"(TRUE ("stage idle?")) -> ()
  n546 = Bundle By Name(cluster=w471, "pipette template"=w469, "pipette mask for cell tracker"=w465, "found pipette"=w468) -> (w467:T54)
  n547 = local write "stage reservation options"(w407) -> ()
  n548 = local write "individual controls manip 1"(w246) -> ()
  n549 = local write "individual controls manip 2"(w249) -> ()
  n550 = local read "multiclamp control?"() -> (w699:bool)
  n551 = Open/Create/Replace File(file path (use dialog)=w696) -> (refnum out=w693:refnum<file>, cancelled=w695:bool, error out=w694:errorcluster)  [unwired: 5 in]
  n552 = case shown="False" w695 {
    tunnel: w694 -> [w756 _]
    tunnel: w693 -> [w755 _]
    frame False {
      # "load default locations"
      n553 = local read "mock location array"() -> (w757:dbl[][])
      n554 = Read from Text File(file (use dialog)=w755, error in=w756) -> (refnum out=w760:refnum<file>, text=w761:string, error out=w762:errorcluster)  [unwired: 2 in, 1 out]
      n555 = Unflatten From String(type=w757, binary string=w761, error in (no error)=w762) -> (value=w758:dbl[][], error out=w759:errorcluster)  [unwired: 2 in, 1 out]
      n556 = Index Array(array=w758) -> (element #1=w741:dbl[], element #2=w740:dbl[], element #3=w739:dbl[], element #4=w738:dbl[], element #5=w737:dbl[], element #6=w736:dbl[], element #7=w754:dbl[], element #8=w753:dbl[], element #9=w752:dbl[], element #10=w751:dbl[], element #11=w750:dbl[], element #12=w749:dbl[], element #13=w748:dbl[], element #14=w747:dbl[], element #15=w746:dbl[], element #16=w745:dbl[], element #17=w744:dbl[], element #18=w743:dbl[], element #19=w742:dbl[])  [unwired: 38 in]
      n557 = Close File(refnum=w760, error in=w759) -> ()  [unwired: 2 out]
      n558 = local write "Jumper Position o-C"(w754) -> ()
      n559 = local write "Jumper Position C-o"(w753) -> ()
      n560 = local write "Jumper Position C-B"(w752) -> ()
      n561 = local write "Jumper Position B-C"(w751) -> ()
      n562 = local write "Jumper Position B-A"(w750) -> ()
      n563 = local write "Jumper Position A-B"(w749) -> ()
      n564 = local write "Jumper Position A-o"(w748) -> ()
      n565 = local write "Jumper Position o-A"(w747) -> ()
      n566 = local write "Jumper Position C"(w746) -> ()
      n567 = local write "Jumper Position B"(w745) -> ()
      n568 = local write "Jumper Position A"(w744) -> ()
      n569 = local write "Experiment Safe Position"(w743) -> ()
      n570 = local write "Jumper Safe Position"(w742) -> ()
      n571 = local write "cleaning bath loc 1"(w740) -> ()
      n572 = local write "loc above baths 1"(w741) -> ()
      n573 = local write "loc above baths 2"(w738) -> ()
      n574 = local write "cleaning bath loc 2"(w737) -> ()
      n575 = local write "wash bath loc 2"(w736) -> ()
      n576 = local write "wash bath loc 1"(w739) -> ()
    }
    frame True {
    }
  }
  n577 = local read "holding V (mV)"() -> (w250:dbl)
  n578 = local read "manip1->cam"() -> (w255:T25)
  n579 = local read "manip2->cam"() -> (w256:T25)
  n580 = Bundle By Name(cluster=w255, "zero loc (x,y,z)"=w536) -> (w634:T25)
  n581 = Bundle By Name(cluster=w256, "zero loc (x,y,z)"=w536) -> (w535:T25)
  n582 = control-ref of="Command pressure (mBar) 2"() -> (w483:refnum<vi>)
  n583 = control-ref of="Command pressure (mBar) 1"() -> (w684:refnum<vi>)
  n584 = local read "pressure box 1"() -> (w260:T14)
  n585 = local write "manip2->cam"(w535) -> ()
  n586 = Unbundle By Name(w535) -> ("actuator"=w534:T26)
  n587 = case shown="True" w699 {
    tunnel: [w766 0] -> w671
    tunnel: [w765 w768] -> w672
    tunnel: [errorcluster {"status"=FALSE, "code"=0, "source"=""} ("error out") w771] -> w698
    tunnel: w250 -> [_ w770]
    frame False {
      w764 = u32 0 ("Multiclamp Handle Out")
      # "irrelevant"
      n588 = To Unsigned Long Integer(number=w764) -> (unsigned 32bit integer=w765:u32)
      n589 = To Long Integer(number=w764) -> (32bit integer=w766:i32)
    }
    frame True {
      n590 = local read "channels to initialize"() -> (w767:T31)
      n591 = call "init multiclamp_N.vi"("channels to initialize"=w767, "holding V (mV)"=w770) -> ("error out"=w771:errorcluster, "mclamp cluster out"=w769:T30, "Multiclamp Handle Out"=w768:u32)  [unwired: 6 in, 1 out]
      n592 = local write "mclamp cluster"(w769) -> ()
      n593 = local write "Multiclamp Handle"(w768) -> ()
    }
  }
  n594 = Unbundle By Name(w634) -> ("actuator"=w653:T26)
  n595 = local write "manip1->cam"(w634) -> ()
  n596 = call "initPressure_topLvl.vi"("Pressure box control in"=w260) -> ("error out"=w685:errorcluster, "Pressure box control out"=w686:T14)  [unwired: 9 in]
  n597 = local read "stage->cam"() -> (w257:T25)
  n598 = call "switchPressure_topLvl.vi"("which manipulator"=w444, "Slide Refnum"=w684, "error in"=w685, "pressure setting"=w474, "Pressure box control in"=w686) -> ("error out"=w449:errorcluster, "Pressure box control out"=w448:T14)  [unwired: 5 in]
  n599 = control-ref of="manip3->cam"() -> (w655:refnum<vi>)
  n600 = control-ref of="manip2->cam"() -> (w657:refnum<vi>)
  n601 = control-ref of="manip4->cam"() -> (w654:refnum<vi>)
  n602 = control-ref of="stage->cam"() -> (w658:refnum<vi>)
  n603 = control-ref of="manip1->cam"() -> (w656:refnum<vi>)
  n604 = Unbundle By Name(w257) -> ("actuator"=w429:T26)
  n605 = call "switchSolenoid_topLvl.vi"("which manipulator"=w444, "error in (no error)"=w449, "solenoidSwitch (T:atm; F: Reg)"=FALSE, "Pressure box control in"=w448) -> ("error out"=w446:errorcluster, "Pressure box control out"=w447:T14)  [unwired: 6 in]
  n606 = Get Date/Time In Seconds() -> (seconds since 1Jan1904=w520:timestamp)
  n607 = call "init manipulator.vi"("Actuator cluster in"=w534) -> ("error out"=w533:errorcluster, "Actuator cluster out"=w338:T26)  [unwired: 7 in, 2 out]
  n608 = call "init manipulator.vi"("Actuator cluster in"=w653) -> ("error out"=w687:errorcluster, "Actuator cluster out"=w378:T26)  [unwired: 7 in, 2 out]
  n609 = local read "temp pipette 2 template location"() -> (w269:path)
  n610 = control-ref of="current stage pos (steps)"() -> (w692:refnum<vi>)
  n611 = control-ref of="current manip 1 pos (steps)"() -> (w691:refnum<vi>)
  n612 = control-ref of="current manip 2 pos (steps)"() -> (w690:refnum<vi>)
  n613 = control-ref of="current manip 3 pos (steps)"() -> (w689:refnum<vi>)
  n614 = control-ref of="current manip 4 pos (steps)"() -> (w688:refnum<vi>)
  n615 = call "IMAQ Create"("Border Size"=0, "Image Name"="view", "Image Type"=w332) -> ("New Image"=w366:T10, "error out"=w333:errorcluster)  [unwired: 2 in]
  n616 = call "IMAQ Create"("Border Size"=0, "Image Name"="orig", "Image Type"=w332) -> ("New Image"=w276:T10)  [unwired: 2 in, 1 out]
  n617 = call "init stage.vi"("stage motion"=scope_motion."slow_dualPatch", "Actuator cluster in"=w429) -> ("Actuator cluster out"=w336:T26)  [unwired: 7 in, 2 out]
  n618 = call "switchPressure_topLvl.vi"("which manipulator"=w440, "Slide Refnum"=w483, "error in"=w446, "pressure setting"=w474, "Pressure box control in"=w447) -> ("error out"=w442:errorcluster, "Pressure box control out"=w443:T14)  [unwired: 5 in]
  n619 = Not Equal To 0?(x=w671) -> (x != 0?=w673:bool)
  n620 = local read "temp pipette 1 template location"() -> (w265:path)
  n621 = Bundle By Name(cluster=T36 {"s"=refnum, "manip 1"=refnum, "manip 2"=refnum, "manip 3"=refnum, "manip 4"=refnum} ("transform cluster + actuator"), "s"=w658, "manip 1"=w656, "manip 2"=w657, "manip 3"=w655, "manip 4"=w654) -> (w272:T36)
  n622 = local read "Valve1 Connected"() -> (w286:bool)
  n623 = Bundle("current stage pos (steps)"=w692, "current manip 1 pos (steps)"=w691, "current manip 2 pos (steps)"=w690, "current manip 3 pos (steps)"=w689, "current manip 4 pos (steps)"=w688) -> (w270:T35)  [unwired: 1 in]
  n624 = call "switchSolenoid_topLvl.vi"("which manipulator"=w440, "error in (no error)"=w442, "solenoidSwitch (T:atm; F: Reg)"=FALSE, "Pressure box control in"=w443) -> ("error out"=w441:errorcluster, "Pressure box control out"=w322:T14)  [unwired: 6 in]
  n625 = local read "pipette 1 mask"() -> (w264:path)
  n626 = local read "P1 state"() -> (w364:T11)
  n627 = Format Into String(w518) -> (resulting string=w519:string)  [unwired: 3 in, 1 out]
  n628 = local read "P1 state"() -> (w361:T11)
  n629 = Format Into String(w518) -> (resulting string=w700:string)  [unwired: 3 in, 1 out]
  n630 = local write "orig image"(w276) -> ()
  n631 = local write "Slice view"(w276) -> ()
  n632 = call "IMAQ Create"("Image Name"="pipette 1 template", "Image Type"=w433) -> ("New Image"=w632:T10)  [unwired: 3 in, 1 out]
  n633 = call "IMAQ Create"("Image Name"="pipette mask 1", "Image Type"=w365) -> ("New Image"=w628:T10)  [unwired: 3 in, 1 out]
  n634 = call "IMAQ Create"("Image Name"="pipette 2 corrMask", "Image Type"=w365) -> ("New Image"=w431:T10)  [unwired: 3 in, 1 out]
  n635 = call "IMAQ Create"("Image Name"="pipette 1 corrMask", "Image Type"=w365) -> ("New Image"=w432:T10)  [unwired: 3 in, 1 out]
  n636 = local write "transforms"(w272) -> ()
  n637 = Not Equal?(x=w364, y=user_message_v6."Setting defaults..." ("P1 state")) -> (x != y?=w360:bool)
  n638 = call "IMAQ Create"("Image Name"="pipette mask 2", "Image Type"=w365) -> ("New Image"=w463:T10)  [unwired: 3 in, 1 out]
  n639 = call "IMAQ Create"("Image Name"="pipette 1 mask for cell tracker", "Image Type"=w433) -> ("New Image"=w456:T10)  [unwired: 3 in, 1 out]
  n640 = call "IMAQ Create"("Image Name"="pipette 2 template", "Image Type"=w433) -> ("New Image"=w460:T10)  [unwired: 3 in, 1 out]
  n641 = Not Equal?(x=w361, y=user_message_v6."Initializing..." ("P1 state")) -> (x != y?=w359:bool)
  n642 = call "multiclamp error"("Enable"=w673) -> ()  [unwired: 9 in, 2 out]
  n643 = call "IMAQ Create"("Image Name"="pipette 1 mask for cell tracker", "Image Type"=w433) -> ("New Image"=w621:T10)  [unwired: 3 in, 1 out]
  n644 = Build Array(w519) -> (w254:string[])
  n645 = local read "3D Graph"() -> (w271:refnum<k7>)
  n646 = Build Array(w700) -> (w252:string[])
  n647 = local read "camera type"() -> (w277:T22)
  n648 = local write "positions"(w270) -> ()
  n649 = local write "state list manip 1"(w252) -> ()
  n650 = Or(x=w360, y=w359) -> (x .or. y?=w288:bool)
  n651 = Select(t=w288, s=w286, f=w286) -> (s? t:f=w287:bool)
  n652 = local read "pipette 2 mask"() -> (w268:path)
  n653 = local write "state list manip 2"(w254) -> ()
  n654 = call "IMAQ ReadFile"("File Path"=w265, "Image"=w632) -> ("error out"=w629:errorcluster, "Image Out"=w630:T10)  [unwired: 5 in, 3 out]
  n655 = call "IMAQ ReadFile"("File Path"=w269, "Image"=w460) -> ("error out"=w459:errorcluster, "Image Out"=w458:T10)  [unwired: 5 in, 3 out]
  n656 = call "IMAQ ReadFile"("File Path"=w264, "Image"=w628) -> ("Image Out"=w627:T10)  [unwired: 5 in, 4 out]
  n657 = local read "manip 1 on"() -> (w251:bool)
  n658 = Merge Errors(w698, w687, w441, w533, w279) -> (w278:errorcluster)
  n659 = local read "manip 2 on"() -> (w253:bool)
  n660 = call "IMAQ ReadFile"("File Path"=w268, "Image"=w463) -> ("Image Out"=w464:T10)  [unwired: 5 in, 4 out]
  n661 = call "IMAQ Learn Pattern 5"("Image"=w630, "Algorithm"=w631, "Mask"=w627, "error in (no error)"=w629) -> ("Template Image Out"=w266:T10)  [unwired: 9 in, 2 out]
  n662 = call "IMAQ Learn Pattern 5"("Image"=w458, "Algorithm"=w457, "Mask"=w464, "error in (no error)"=w459) -> ("Template Image Out"=w267:T10)  [unwired: 9 in, 2 out]
  n663 = Unbundle By Name(w278) -> ("status"=w703:bool)
  n664 = local write "pipette 1 template"(w266) -> ()
  n665 = Obtain Notifier(name (unnamed)="Main Stop Notifier", notification data type=FALSE ("stop events")) -> (notifier out=w394:refnum<notifier>, error out=w398:errorcluster)  [unwired: 2 in, 1 out]
  n666 = while {
    tunnel: w398 -> [w834]